vi "HFRR ADV v042.vi"() -> ()   [LabVIEW 2025] (continued)
        n1759 = Not Equal?(x=w2092, y=w2091) -> (x != y?=w2089:bool)
        n1760 = case shown="True" w2097 {
          frame False {
            w2103 = TRUE ("Visible")
            n1761 = property on="Port 1a" class="Bool (strict)"("Visible"=w2103) -> ()  [unwired: 2 in, 2 out]
            n1762 = property on="Port 3" class="Bool (strict)"("Visible"=w2103) -> ()  [unwired: 2 in, 2 out]
          }
          frame True {
            w2104 = TRUE ("Visible")
            n1763 = property on="Port 1a" class="Bool (strict)"("Visible"=w2104) -> ()  [unwired: 2 in, 2 out]
            n1764 = property on="Port 3" class="Bool (strict)"("Visible"=w2104) -> ()  [unwired: 2 in, 2 out]
          }
        }
        n1765 = Wait (ms)(milliseconds to wait=u32 40) -> ()  [unwired: 1 out]
        n1766 = case shown="True" w2089 {
          tunnel: [w2101 errorcluster {"status"=TRUE, "code"=0, "source"="Init"} ("error out")] -> w2090
          tunnel: w2093 -> [w2101 _]
          frame False {
          }
          frame True {
          }
        }
        n1767 = case shown="Error" w2090 {
          selector: w2090 -> [w2111 w2129]
          tunnel: [w2114 w2133] -> w2100
          tunnel: [w2113 w2127] -> w2099
          tunnel: w2091 -> [w2112 w2131]
          frame No Error {
            n1768 = property class="Instr"(reference=w2112, error in=w2111) -> (reference out=w2109:refnum<visa-resource-name>, error out=w2110:errorcluster, "Serial Settings:Number of Bytes at Serial Port"=w2106:u32)
            n1769 = Greater?(x=w2106, y=u32 5) -> (0:w2105:bool)
            n1770 = Not(x=w2105) -> (.not. x?=→"Port 1a":bool)
            n1771 = while {
              tunnel: [w2122] -> w2113
              tunnel: [w2121] -> w2114
              tunnel: w2110 -> [w2120]
              tunnel: w2109 -> [w2119]
              stop <- TRUE stop-if-true
              n1772 = property class="Instr" props=["Serial Settings:Number of Bytes at Serial Port"](reference=w2119, error in=w2120) -> (reference out=w2124:refnum<visa-resource-name>, error out=w2123:errorcluster)  [unwired: 1 out]
              n1773 = VISA Read(VISA resource name=w2124, byte count=u32 50, error in (no error)=w2123) -> (VISA resource name out=w2121:refnum<visa-resource-name>, read buffer=w2116:string, error out=w2122:errorcluster)  [unwired: 1 out]
              n1774 = Wait (ms)(milliseconds to wait=u32 5) -> ()  [unwired: 1 out]
            }
          }
          frame Error {
            w2139 = u16 0 items=["None", "XON/XOFF", "RTS/CTS", "XON/XOFF & RTS/CTS", "DTR/DSR", "XON/XOFF & DTR/DSR"] ("flow control (0:none)  2")
            w2137 = u16 10 items=["1.0"=10, "1.5"=15, "2.0"=20] ("stop bits 2")
            w2135 = u16 0 items=["None", "Odd", "Even", "Mark", "Space"] ("parity 2")
            w2136 = u32 10000  # timeout (10sec)
            n1775 = VISA Close(VISA resource name=w2131, error in (no error)=w2129) -> (error out=w2132:errorcluster)
            n1776 = local write "Port 1a"(FALSE ("Port 1a")) -> ()
            n1777 = local read "Com Port 1"() -> (w2126:refnum<visa-resource-name>)
            n1778 = call <vilib>:"Clear Errors.vi"("error in (no error)"=w2132) -> ("error out"=w2130:errorcluster)  [unwired: 5 in, 1 out]
            n1779 = call-poly "VISA Configure Serial Port"("VISA resource name"=w2126, "timeout (10sec)"=w2136, "baud rate (9600)"=u32 250000 ("baud rate  2"), "data bits (8)"=u16 8 ("data bits  2"), "parity (0:none)"=w2135, "error in (no error)"=w2130, "stop bits (10: 1 bit)"=w2137, "flow control (0:none)"=w2139) -> ("VISA resource name out"=w2140:refnum<visa-resource-name>, "error out"=w2141:errorcluster)  [unwired: 6 in]
            n1780 = flat-sequence {
              tunnel: w2140 -> [w2143]
              tunnel: w2141 -> [w2142]
              tunnel: [w2143] -> w2133
              tunnel: [w2142] -> w2127
              frame #0 {
                n1781 = Wait (ms)(milliseconds to wait=u32 50) -> ()  [unwired: 1 out]
              }
            }
            "Residual Uno" <- ""
          }
        }
        n1782 = local read "Quit"() -> (w2088:bool)
        "Error Uno" <- w2093
      }
      n1783 = VISA Close(VISA resource name=w2086, error in (no error)=w2085) -> (error out=w2083:errorcluster)
      n1784 = call <vilib>:"Clear Errors.vi"("error in (no error)"=w2083) -> ()  [unwired: 5 in, 2 out]
    }
    frame Enabled {
    }
  }
  n1785 = while {
    stop <- w2154 stop-if-true
    # "V0OLTAGE TO STROKE (peice vise calibration)"
    n1786 = local read "LVDT MIN"() -> (w2146:dbl)
    n1787 = local read "LVDT Peak"() -> (w2145:dbl)
    n1788 = Wait (ms)(milliseconds to wait=u32 10) -> ()  [unwired: 1 out]
    n1789 = formula code="// Dynamic Parameterized Linear Interpolation Node\n// Inputs: vpp_val, voltages (Array), distances (Array)\n// Outputs: stroke\n\nint i = 0;\nint segments = 11; // 12 points make 11 interpolation segments\n\n// 1. Lower Boundary Clamp\nif (vpp_val <= voltages[0]) {\n    stroke = distances[0];\n}\n// 2. Upper Boundary Clamp\nelse if (vpp_val >= voltages[segments]) {\n    stroke = distances[segments];\n}\n// 3. Dynamic Segment Search Loop\nelse {\n    stroke = distances[0]; // Fallback baseline\n    for (i = 0; i < segments; i++) {\n        if (vpp_val >= voltages[i] && vpp_val <= voltages[i+1]) {\n            // Standard linear interpolation formula using array lookups\n            stroke = distances[i] + (vpp_val - voltages[i]) * (distances[i+1] - distances[i]) / (voltages[i+1] - voltages[i]);\n            break; // Segment found, safely exit the loop\n        }\n    }\n}"("vpp_val"=w2145, "voltages"="calibration values", "distances"="STROKE") -> ("stroke"=→"LVDT STROKE":dbl)
    n1790 = local read "Calibration Tare Value"() -> (w2150:dbl)
    n1791 = local read "Calibration Tare"() -> (w2148:bool)
    n1792 = Subtract(x=w2146, y=w2150) -> (x-y=→"LVDT STROKE  Calibration":dbl)
    n1793 = case shown="True" w2148 {
      selector: w2148 -> [_ w2156]
      tunnel: w2146 -> [_ w2157]
      frame False {
      }
      frame True {
        n1794 = Not(x=w2156) -> (.not. x?=w2155:bool)
        n1795 = local write "Calibration Tare"(w2155) -> ()
        "Calibration Tare Value" <- w2157
      }
    }
    n1796 = local read "Quit"() -> (w2154:bool)
  }
  n1797 = while {
    stop <- w2180 stop-if-true
    n1798 = local read "Due read"() -> (w2178:string)
    n1799 = call <vilib>:"High Resolution Polling Wait.vi"("seconds to wait"=0.02) -> ()  [unwired: 10 in, 1 out]
    n1800 = local read "Frictioin Force Raw"() -> (w2160:dbl)
    n1801 = Spreadsheet String To Array(delimiter (Tab)=";", format string="", spreadsheet string=w2178, array type (2D Dbl)=string[] []) -> (array=w2175:string[])
    n1802 = Fract/Exp String To Number(string=w2175) -> (number=w2174:dbl[])  [unwired: 3 in, 1 out]
    n1803 = call <vilib>:"Median Filter PtByPt.vi"("rank"=2, "x"=w2160) -> ("Filtered x"=→"Friction":dbl)  [unwired: 2 in, 1 out]
    n1804 = Index Array(array=w2174) -> (element #1=→"Sample Temperature":dbl, element #2=→"Target Sample Temperature":dbl, element #3=→"Current Duty Cycle":dbl, element #4=→"Ambient Temperature":dbl, element #5=→"Dac Status":dbl, element #6=→"Vpp":dbl, element #7=→"Active Error Code":dbl, element #8=→"Kp":dbl, element #9=→"Ki":dbl, element #10=→"Kd":dbl, element #11=→"SampleRaw":dbl, element #12=→"AmbRaw":dbl)  [unwired: 12 in]
    n1805 = local read "Quit"() -> (w2180:bool)
  }
  n1806 = while {
    shift-right: [w2194] -> w43
    shift-left: _ -> [w2186]
    shift-right: [w2181] -> w42
    shift-left: errorcluster {"status"=FALSE, "code"=0, "source"="Init"} ("error out") -> [w2188]
    tunnel: [w2183] -> w46
    tunnel: [w2193] -> _
    i -> [w2193]
    stop <- w2183 stop-if-true
    n1807 = local read "Com Port 2"() -> (w2187:refnum<visa-resource-name>)
    n1808 = local read "Port 2a"() -> (w2189:bool)
    n1809 = Unbundle(w2188) -> ("status"=→"Port 4":bool)  [unwired: 2 out]
    n1810 = call <vilib>:"High Resolution Polling Wait.vi"("seconds to wait"=0.02) -> ()  [unwired: 10 in, 1 out]
    n1811 = local read "Port 4"() -> (w2190:bool)
    n1812 = Not Equal?(x=w2187, y=w2186) -> (x != y?=w2185:bool)
    n1813 = Or(x=w2190, y=w2189) -> (x .or. y?=w2192:bool)
    n1814 = case shown="False" w2192 {
      frame False {
        w2197 = TRUE ("Visible")
        n1815 = property on="Port 2a" class="Bool (strict)"("Visible"=w2197) -> ()  [unwired: 2 in, 2 out]
        n1816 = property on="Port 4" class="Bool (strict)"("Visible"=w2197) -> ()  [unwired: 2 in, 2 out]
      }
      frame True {
        w2198 = TRUE ("Visible")
        n1817 = property on="Port 2a" class="Bool (strict)"("Visible"=w2198) -> ()  [unwired: 2 in, 2 out]
        n1818 = property on="Port 4" class="Bool (strict)"("Visible"=w2198) -> ()  [unwired: 2 in, 2 out]
      }
    }
    n1819 = case shown="True" w2185 {
      tunnel: [w2195 errorcluster {"status"=TRUE, "code"=0, "source"="Init"} ("error out")] -> w2184
      tunnel: w2188 -> [w2195 _]
      frame False {
      }
      frame True {
      }
    }
    n1820 = case shown="No Error" w2184 {
      selector: w2184 -> [w2211 w2242]
      tunnel: [w2204 w2247] -> w2194
      tunnel: [w2212 w2240] -> w2181
      tunnel: w2186 -> [w2213 w2245]
      frame No Error {
        n1821 = property class="Instr" props=["Serial Settings:Number of Bytes at Serial Port"](reference=w2213, error in=w2211) -> (reference out=w2205:refnum<visa-resource-name>, error out=w2210:errorcluster)  [unwired: 1 out]
        n1822 = while {
          tunnel: [w2221] -> w2206
          tunnel: [w2220] -> w2207
          tunnel: w2210 -> [w2219]
          tunnel: w2205 -> [w2218]
          tunnel: [w2217] -> _
          i -> [w2217]
          stop <- TRUE stop-if-true
          n1823 = property class="Instr" props=["Serial Settings:Number of Bytes at Serial Port"](reference=w2218, error in=w2219) -> (reference out=w2223:refnum<visa-resource-name>, error out=w2222:errorcluster)  [unwired: 1 out]
          n1824 = VISA Read(VISA resource name=w2223, byte count=u32 1000, error in (no error)=w2222) -> (VISA resource name out=w2220:refnum<visa-resource-name>, read buffer=→"Due read":string, error out=w2221:errorcluster)  [unwired: 1 out]
        }
        n1825 = local read "Due Write"() -> (w2203:string)
        n1826 = call <vilib>:"Trim Whitespace.vi"("string"=w2203) -> ("trimmed string"=w2202:string)  [unwired: 1 in]
        n1827 = Not Equal?(x=w2202, y="") -> (x != y?=w2208:bool)
        n1828 = VISA Flush I/O Buffer(VISA resource name=w2207) -> (VISA resource name out=w2200:refnum<visa-resource-name>, error out=→"error out 10":errorcluster)  [unwired: 2 in]
        n1829 = case shown="True" w2208 {
          tunnel: w2200 -> [w2225 w2230]
          tunnel: [w2225 w2234] -> w2204
          tunnel: w2206 -> [w2224 w2229]
          tunnel: [w2224 w2232] -> w2212
          tunnel: w2202 -> [_ w2228]
          tunnel: [_ w2231] -> _
          frame False {
            # "DATA  WRITE LOOP"
          }
          frame True {
            n1830 = Concatenate Strings(w2228, "\r\n") -> (w2227:string)
            n1831 = VISA Write(VISA resource name=w2230, write buffer=w2227, error in (no error)=w2229) -> (VISA resource name out=w2234:refnum<visa-resource-name>, return count=w2231:u32, error out=w2233:errorcluster)
            n1832 = flat-sequence {
              tunnel: w2233 -> [w2236]
              tunnel: [w2236] -> w2232
              frame #0 {
                n1833 = local write "Due Write"("" ("Command")) -> ()
                n1834 = Wait (ms)(milliseconds to wait=u32 5) -> ()  [unwired: 1 out]
              }
            }
          }
        }
        "Port 2a" <- TRUE ("Port 2a")
      }
      frame Error {
        w2253 = u16 0 items=["None", "XON/XOFF", "RTS/CTS", "XON/XOFF & RTS/CTS", "DTR/DSR", "XON/XOFF & DTR/DSR"] ("flow control (0:none)  2")
        w2251 = u16 10 items=["1.0"=10, "1.5"=15, "2.0"=20] ("stop bits 2")
        w2249 = u16 0 items=["None", "Odd", "Even", "Mark", "Space"] ("parity 2")
        w2250 = u32 10000  # timeout (10sec)
        n1835 = VISA Clear(VISA resource name=w2245, error in (no error)=w2242) -> (VISA resource name out=w2244:refnum<visa-resource-name>, error out=w2243:errorcluster)
        n1836 = VISA Close(VISA resource name=w2244, error in (no error)=w2243) -> (error out=w2246:errorcluster)
        n1837 = call <vilib>:"Clear Errors.vi"("error in (no error)"=w2246) -> ()  [unwired: 5 in, 2 out]
        n1838 = local write "Port 2a"(FALSE ("Port 2a")) -> ()
        n1839 = local read "Com Port 2"() -> (w2239:refnum<visa-resource-name>)
        "visa due" <- w2239
        n1840 = call-poly "VISA Configure Serial Port"("VISA resource name"=w2239, "timeout (10sec)"=w2250, "baud rate (9600)"=u32 250000 ("baud rate  2"), "data bits (8)"=u16 8 ("data bits  2"), "parity (0:none)"=w2249, "stop bits (10: 1 bit)"=w2251, "flow control (0:none)"=w2253) -> ("VISA resource name out"=w2254:refnum<visa-resource-name>, "error out"=w2255:errorcluster)  [unwired: 7 in]
        n1841 = flat-sequence {
          tunnel: w2254 -> [w2257]
          tunnel: w2255 -> [w2256]
          tunnel: [w2257] -> w2247
          tunnel: [w2256] -> w2240
          frame #0 {
            n1842 = Wait (ms)(milliseconds to wait=u32 50) -> ()  [unwired: 1 out]
          }
        }
        "Residual Due" <- ""
      }
    }
    "error out 9" <- w2181
    n1843 = local read "Quit"() -> (w2183:bool)
    "Error Due" <- w2188
  }
  n1844 = local write "FRICVALZ"(0.0 ("FRICVALZ")) -> ()
  n1845 = property on="RUN" class="Bool (strict)"("Visible"=TRUE) -> ()  [unwired: 2 in, 2 out]
  n1846 = while {
    tunnel: [w2272] -> _
    tunnel: [w2259] -> w56
    i -> [w2272]
    stop <- w2259 stop-if-true
    n1847 = local read "conststatus"() -> (w2263:dbl)
    n1848 = local read "Main Tab"() -> (w2261:T2)
    n1849 = local read "EDIT"() -> (w2278:bool)
    n1850 = local read "Rate"() -> (w2277:dbl)
    n1851 = case shown="True" w2278 {
      tunnel: [FALSE TRUE] -> _
      frame False {
      }
      frame True {
      }
    }
    n1852 = Equal?(x=w2261, y=T28."About" ("Main Tab")) -> (x = y?=w2270:bool)
    n1853 = Equal?(x=w2263, y=0.0) -> (x = y?=w2264:bool)
    n1854 = Divide(x=1.0, y=w2277) -> (x/y=w2273:dbl)
    "Time 2" <- w2273
    n1855 = case shown="True" w2264 {
      frame False {
      }
      frame True {
        # "C:\\WinDucom\\calibrate WO 2391.dcf"
        n1856 = local write "Lan flag"(22) -> ()
        n1857 = local write "conststatus"(10.0 ("rpm value : 2")) -> ()
        n1858 = String To Path(string="C:\\LAB-IQ\\calibrate WO 2465.dcf") -> (path=w2284:path)
        n1859 = Open/Create/Replace File "Open File"(file path (use dialog)=w2284) -> (refnum out=w2282:refnum<file>)  [unwired: 5 in, 2 out]
        n1860 = for {
          N: 23 -> [_]
          tunnel: w2282 -> [w2293]
          i -> [w2287]
          (unwired) TRUE ("line mode (F)")
          n1861 = Read from Text File "Read File"(file (use dialog)=w2293) -> (text=w2292:string)  [unwired: 3 in, 3 out]
          n1862 = Match Pattern(string=w2292, regular expression="]") -> (after substring=w2290:string)  [unwired: 1 in, 3 out]
          n1863 = String Subset(string=w2292, offset (0)=5, length (rest)=10 ("length (rest)")) -> (substring=w2285:string)
          n1864 = Fract/Exp String To Number(string=w2285) -> (number=w2286:dbl)  [unwired: 3 in, 1 out]
          n1865 = Match Pattern(string=w2290, regular expression="-") -> (before substring=w2288:string)  [unwired: 1 in, 3 out]
          n1866 = case shown="10" w2287 {
            tunnel: w2286 -> [_ _ _ _ _ _ _ _ _ _ w2300 _ _ _ _ _ _ _ _ _ _ _ _ _]
            tunnel: w2288 -> [_ _ _ _ w2296 w2297 w2298 _ _ _ _ _ _ _ _ _ _ _ _ _ w2301 w2302 w2303 _]
            frame 0 {
            }
            frame 1 {
            }
            frame 2 {
            }
            frame 3 {
            }
            frame 4 {
              n1867 = local write "Com Port 1"(w2296) -> ()
            }
            frame 5 {
              n1868 = local write "Com Port 2"(w2297) -> ()
              n1869 = local write "visa due"(w2297) -> ()
            }
            frame 6 {
              n1870 = String To Path(string=w2298) -> (path=w2299:path)
              n1871 = local write "File Path"(w2299) -> ()
              "String" <- w2298
            }
            frame 7 {
            }
            frame 8 {
            }
            frame 9 {
            }
            frame 10 {
              n1872 = local write "Language Selection"(w2300) -> ()
            }
            frame 11 {
            }
            frame 12 {
            }
            frame 13 {
            }
            frame 14 {
            }
            frame 15 {
            }
            frame 16 {
            }
            frame 17 {
            }
            frame 18 {
            }
            frame 21 {
            }
            frame 22 {
              n1873 = local write "Com Port 3"(w2301) -> ()
            }
            frame 20 {
              n1874 = local write "Camera Port :"(w2302) -> ()
            }
            frame 19 {
              n1875 = local write "C3 :"(w2303) -> ()
            }
            frame 23, Default {
            }
          }
        }
      }
    }
    n1876 = Select(t=u32 2500 ("milliseconds to wait"), s=w2270, f=u32 500 ("milliseconds to wait")) -> (s? t:f=w2268:u32)
    n1877 = Multiply(x=w2273, y=w2268) -> (x*y=w2275:dbl)
    n1878 = call "Elapsed Time2"("Time Target (s)"=w2275, "Auto Reset"=TRUE) -> ("Time has Elapsed"=w2265:bool)  [unwired: 10 in, 7 out]
    n1879 = case shown="True" w2265 {
      frame False {
      }
      frame True {
        n1880 = stacked-sequence {
          frame #0 {
            # "DATA PROCESSING"
            # "115 mV/N"
            n1881 = local read "Sample Temperature"() -> (w2306:dbl)
            n1882 = local read "RH Numeric:"() -> (→"Humidity ( %RH )":dbl)
            n1883 = local read "FRICVALZ"() -> (w2323:dbl)
            n1884 = local read "Friction"() -> (w2309:dbl)
            n1885 = call <vilib>:"Mean PtByPt.vi"("x"=w2306, "sample length"=100) -> ("mean"=w2305:dbl)  [unwired: 2 in, 1 out]
            "TEMP 2" <- w2305
            "TEMP 3" <- w2305
            n1886 = Subtract(x=w2309, y=w2323) -> (x-y=w2318:dbl)
            "FF 2" <- w2318
            "FF 4" <- w2318
            n1887 = local read "Ambient Temperature"() -> (→"AIR TEMP":dbl)
            n1888 = local read "TEMP"() -> (w2322:dbl)
            n1889 = local write "FF 3"(w2318) -> ()
            n1890 = Compound Arithmetic op=OR("FRICVALZ 4", "FRICVALZ 3", "FRICVALZ 2") -> (w2314:bool)
            n1891 = case shown="True" w2314 {
              tunnel: w2309 -> [_ w2329]
              frame False {
              }
              frame True {
                w2328 = FALSE ("FRICVALZ")
                n1892 = local write "FRICVALZ 3"(w2328) -> ()
                n1893 = local write "FRICVALZ 2"(w2328) -> ()
                n1894 = local write "FRICVALZ 4"(w2328) -> ()
                "FRICVALZ" <- w2329
              }
            }
            n1895 = Not A Number/Path/Refnum?(number/path/refnum=w2322) -> (NaN/Path/Refnum?=w2321:bool)
            n1896 = Not A Number/Path/Refnum?(number/path/refnum=w2318) -> (NaN/Path/Refnum?=w2320:bool)
            n1897 = Divide(x=w2318, y=1.96) -> (x/y=w2315:dbl)
            n1898 = Compound Arithmetic op=OR(w2321, w2320) -> (w2319:bool)
            n1899 = Not A Number/Path/Refnum?(number/path/refnum=w2315) -> (NaN/Path/Refnum?=w2316:bool)
            n1900 = case shown="True" w2319 {
              frame False {
              }
              frame True {
                n1901 = local write "TEMP"(0.0 ("TEMP")) -> ()
                n1902 = local write "FF 2"(0.0 ("FF 2")) -> ()
                n1903 = local write "reinit"(TRUE ("reinit")) -> ()
              }
            }
            n1904 = local write "TEMP"(w2305) -> ()
            n1905 = Select(t=0.0, s=w2316, f=w2315) -> (s? t:f=w2308:dbl)
            "COF 2" <- w2308
            n1906 = local write "COF 3"(w2308) -> ()
          }
        }
      }
    }
    n1907 = Wait (ms)(milliseconds to wait=u32 50) -> ()  [unwired: 1 out]
    n1908 = local read "Quit"() -> (w2259:bool)
    "Rate" <- 2500.0 ("No of Samples")
  }
  n1909 = while {
    tunnel: [w2349] -> _
    tunnel: [w2332] -> w58
    tunnel: w3 -> [_]
    i -> [w2349]
    stop <- w2332 stop-if-true
    # "C:\\LAB-IQ-NXT\\Scar View.exe"
    n1910 = local read "OK Button 16"() -> (w2339:bool)
    n1911 = local read "Main Tab"() -> (w2333:T2)
    n1912 = local read "service 3"() -> (w2334:bool)
    n1913 = local read "OPEN 6"() -> (w2336:bool)
    n1914 = local read "EDIT 2"() -> (w2338:bool)
    n1915 = flat-sequence {
      frame #0 {
        n1916 = stacked-sequence {
          frame #0 {
            n1917 = local read "EDIT"() -> (w2827:bool)
            n1918 = case shown="False" w2827 {
              tunnel: [u8 2 ("Disabled") u8 0 ("Disabled")] -> _
              frame False {
                w2829 = FALSE
                n1919 = local write "Password"("") -> ()
                n1920 = local write "x = y?"(w2829) -> ()
                n1921 = property on="Password" class="Str"("Visible"=w2829) -> ()  [unwired: 2 in, 2 out]
              }
              frame True {
                n1922 = property on="Password" class="Str"("Visible"=TRUE) -> ()  [unwired: 2 in, 2 out]
              }
            }
            "dipl pwd" <- "@143$\n" ("dipl pwd")
          }
          frame #1 {
          }
          frame #2 {
          }
          frame #3 {
          }
          frame #4 {
            n1923 = String To Byte Array(string="Password") -> (unsigned byte array=w2840:u8[])
            n1924 = Search 1D Array(1D array=w2840, element=u8 10) -> (index of element=w2838:i32)  [unwired: 1 in]
            n1925 = Index Array(array=w2840, index=w2838) -> (element=w2839:u8)
            n1926 = Equal?(x=w2839, y=10) -> (x = y?=w2835:bool)
            n1927 = case shown="True" w2835 {
              frame False {
              }
              frame True {
                # "password"
                # "password"
                n1928 = local read "Password"() -> (w2852:string)
                n1929 = String To Byte Array(string=w2852) -> (unsigned byte array=w2855:u8[])
                n1930 = String To Byte Array(string="@143$\n") -> (unsigned byte array=w2842:u8[])
                n1931 = Array Size(array=w2855) -> (size(s)=w2851:i32)
                n1932 = Array Size(array=w2842) -> (size(s)=w2847:i32)
                n1933 = for {
                  N: w2851 -> [_]
                  tunnel: w2855 -> [w2868]
                  tunnel: [w2866] -> w2856 mode=indexing
                  tunnel: w2851 -> [w2863]
                  i -> [w2864]
                  n1934 = Decrement(x=w2863) -> (x-1=w2862:i32)
                  n1935 = Index Array(array=w2868, index=w2864) -> (element=w2867:u8)
                  n1936 = Equal?(x=w2864, y=w2862) -> (x = y?=w2861:bool)
                  n1937 = Number To Decimal String(number=w2867) -> (decimal integer string=w2865:string)  [unwired: 1 in]
                  n1938 = Select(t="", s=w2861, f="\r") -> (s? t:f=w2858:string)
                  n1939 = Concatenate Strings(w2865, w2858) -> (w2866:string)
                }
                n1940 = for {
                  N: w2847 -> [_]
                  tunnel: w2842 -> [w2879]
                  tunnel: [w2877] -> w2845 mode=indexing
                  tunnel: w2847 -> [w2874]
                  i -> [w2875]
                  n1941 = Decrement(x=w2874) -> (x-1=w2873:i32)
                  n1942 = Index Array(array=w2879, index=w2875) -> (element=w2878:u8)
                  n1943 = Equal?(x=w2875, y=w2873) -> (x = y?=w2872:bool)
                  n1944 = Number To Decimal String(number=w2878) -> (decimal integer string=w2876:string)  [unwired: 1 in]
                  n1945 = Select(t="", s=w2872, f="\r") -> (s? t:f=w2869:string)
                  n1946 = Concatenate Strings(w2876, w2869) -> (w2877:string)
                }
                n1947 = local read "file path"() -> (w2841:path)
                n1948 = call <vilib>:"Read Characters From File.vi"("file path (dialog if empty)"=w2841) -> ("character string"=w2854:string)  [unwired: 5 in, 3 out]
                "string" <- w2854
                n1949 = flat-sequence {
                  tunnel: [w2857] -> _
                  frame #0 {
                    w2857 = ""
                    n1950 = local write "Password"(w2857) -> ()
                  }
                }
                n1951 = Concatenate Strings(w2845) -> (w2846:string)
                n1952 = Concatenate Strings(w2854) -> (w2853:string)
                n1953 = Concatenate Strings(w2856) -> (w2849:string)
                n1954 = Equal?(x=w2849, y=w2853) -> (x = y?=w2844:bool)
                n1955 = Equal?(x=w2849, y=w2846) -> (x = y?=w2850:bool)
                n1956 = Or(x=w2844, y=w2850) -> (x .or. y?=→"x = y?":bool)
              }
            }
          }
        }
        n1957 = local read "x = y?"() -> (w2825:bool)
        n1958 = And(x="EDIT", y=w2825) -> (x .and. y?=w2823:bool)
        n1959 = case shown="True" w2823 {
          tunnel: [u8 2 ("Disabled") u8 0 ("Disabled")] -> w2822
          tunnel: [w3029 TRUE ("Visible")] -> w2821
          frame False {
            w3029 = FALSE ("Visible")
            n1960 = local write "EDIT 2"(w3029) -> ()
          }
          frame True {
          }
        }
        n1961 = case shown="True" "SAVE" {
          frame False {
          }
          frame True {
            n1962 = stacked-sequence {
              seq-local: [w2884 _ _] -> [_ w3025 _]
              frame #0 {
                w2880 = 0.0 ("number")
                w2881 = 0.0 ("number")
                (unwired) i16 5 ("precision (6)")
                # "[CH1]    - FF\n[CH2]   - TEMPERATURE\n[CH3]    - Humidity\n[CH4]    - AIR TEMP\n[CH5]\\- Visa Uno\n[CH6] \\- Visa Due\n[CH7]  \\- file path\n[CH8]   - Displacement Gain\n[CHA]   - Stroke Gain\n[CHB]   - Stroke PID Gain\n[CHC]   -Language Selection\n[CHD]   -Power +\n[CHE]   -Power_\n[CHF]   -Heater\n[CHG]   -Humidity Wet\n[CHH]   -Humidity Dry\n[CHI]   -Integral Time"
                n1963 = local read "Language Selection"() -> (w2927:enum16{"English", "Russian"})
                n1964 = Path To String(path="File Path") -> (string=w2943:string)
                n1965 = Number To Fractional String(number=w2880, width (-)=i16 10 ("precision (6)"), precision (6)=i16 5) -> (F-format string=w2934:string)  [unwired: 1 in]
                n1966 = Number To Fractional String(number=w2927, width (-)=i16 10 ("precision (6)"), precision (6)=i16 5) -> (F-format string=w2923:string)  [unwired: 1 in]
                n1967 = Number To Fractional String(number=w2881, width (-)=i16 10 ("precision (6)"), precision (6)=i16 5) -> (F-format string=w2917:string)  [unwired: 1 in]
                n1968 = Number To Fractional String(number=w2881, width (-)=i16 10 ("precision (6)"), precision (6)=i16 5) -> (F-format string=w2914:string)  [unwired: 1 in]
                n1969 = Number To Fractional String(number=w2881, width (-)=i16 10 ("precision (6)"), precision (6)=i16 5) -> (F-format string=w2909:string)  [unwired: 1 in]
                n1970 = Number To Fractional String(number=w2881, width (-)=i16 10 ("precision (6)"), precision (6)=i16 5) -> (F-format string=w2906:string)  [unwired: 1 in]
                n1971 = Number To Fractional String(number=w2881, width (-)=i16 10 ("precision (6)"), precision (6)=i16 5) -> (F-format string=w2901:string)  [unwired: 1 in]
                n1972 = local read "Com Port 1"() -> (w2883:refnum<visa-resource-name>)
                n1973 = local read "Com Port 2"() -> (w2882:refnum<visa-resource-name>)
                n1974 = Concatenate Strings(w2943, "\\" ("string")) -> (w2942:string)
                n1975 = Number To Fractional String(number=w2880, width (-)=i16 10 ("precision (6)"), precision (6)=i16 5) -> (F-format string=w2975:string)  [unwired: 1 in]
                n1976 = Number To Fractional String(number=w2880, width (-)=i16 10 ("precision (6)"), precision (6)=i16 5) -> (F-format string=w2974:string)  [unwired: 1 in]
                n1977 = Number To Fractional String(number=w2880, width (-)=i16 10 ("precision (6)"), precision (6)=i16 5) -> (F-format string=w2968:string)  [unwired: 1 in]
                n1978 = Number To Fractional String(number=w2880, width (-)=i16 10 ("precision (6)"), precision (6)=i16 5) -> (F-format string=w2962:string)  [unwired: 1 in]
                n1979 = Number To Fractional String(number=w2880, width (-)=i16 10 ("precision (6)"), precision (6)=i16 5) -> (F-format string=w2935:string)  [unwired: 1 in]
                n1980 = Concatenate Strings("[CHA]" ("string"), w2934, "- Stroke Gain" ("string"), "\r") -> (w2928:string)
                n1981 = Concatenate Strings("[CHC]" ("string"), w2923, "-Language Selection" ("string"), "\r") -> (w2920:string)
                n1982 = Concatenate Strings("[CHD]" ("string"), w2917, "-Power +" ("string"), "\r") -> (w2899:string)
                n1983 = Concatenate Strings("[CHG]" ("string"), w2906, "-Humidity Wet" ("string"), "\r") -> (w2896:string)
                n1984 = Concatenate Strings("[CHH]" ("string"), w2901, "-Humidity Dry" ("string"), "\r") -> (w2895:string)
                n1985 = Concatenate Strings("[CH1]" ("string"), w2975, " - FF" ("string"), "\r") -> (w2973:string)
                n1986 = Concatenate Strings("[CH2]" ("string"), w2974, " - TEMPERATURE" ("string"), "\r") -> (w2972:string)
                n1987 = Concatenate Strings("[CH3]" ("string"), w2968, " - Humidity" ("string"), "\r") -> (w2965:string)
                n1988 = Concatenate Strings("[CH4]" ("string"), w2962, " - AIR TEMP" ("string"), "\r") -> (w2958:string)
                n1989 = Concatenate Strings("[CH5]" ("string"), w2883, "- Visa Uno" ("string"), "\r") -> (w2951:string)
                n1990 = Concatenate Strings("[CH6]" ("string"), w2882, "- Visa Due" ("string"), "\r") -> (w2946:string)
                n1991 = Concatenate Strings("[CH7]" ("string"), w2942, "- file path" ("string"), "\r") -> (w2945:string)
                n1992 = Concatenate Strings("[CH8]" ("string"), w2935, "- Displacement Gain" ("string"), "\r") -> (w2938:string)
                n1993 = Concatenate Strings("[CHE]" ("string"), w2914, "-Power_" ("string"), "\r") -> (w2898:string)
                n1994 = Concatenate Strings("[CHF]" ("string"), w2909, "-Heater" ("string"), "\r") -> (w2897:string)
                n1995 = Concatenate Strings(w2973, w2972, w2965, w2958, w2951, w2946, w2945, w2938, w2928, w2920, w2899, w2898, w2897, w2896, w2895) -> (w2884:string)
                "gain" <- w2884
              }
              frame #1 {
                w2986 = 0.0 ("number")
                n1996 = local read "Camera Port :"() -> (w2989:string)
                n1997 = local read "C3 :"() -> (w2997:refnum<visa-resource-name>)
                n1998 = local read "Com Port 3"() -> (w2998:refnum<visa-resource-name>)
                n1999 = Concatenate Strings("[CH8]" ("string"), w2989, "- Visa Camera" ("string"), "\r") -> (w2988:string)
                n2000 = Concatenate Strings("[CH7]" ("string"), w2997, "- Visa Humidity" ("string"), "\r") -> (w2993:string)
                n2001 = Number To Fractional String(number=w2986, width (-)=i16 10 ("precision (6)"), precision (6)=i16 5) -> (F-format string=w3013:string)  [unwired: 1 in]
                n2002 = Concatenate Strings("[CHL]" ("string"), w2998, "- Visa humid" ("string"), "\r") -> (w3001:string)
                n2003 = Number To Fractional String(number=w2986, width (-)=i16 10 ("precision (6)"), precision (6)=i16 5) -> (F-format string=w3020:string)  [unwired: 1 in]
                n2004 = Concatenate Strings("[CHK]" ("string"), w3013, "-TEMP INTERCEPT" ("string"), "\r") -> (w3009:string)
                n2005 = Concatenate Strings("[SNO]" ("string"), "" ("string"), "-" ("string"), "\r") -> (w3006:string)
                n2006 = Concatenate Strings("[CHJ]" ("string"), w3020, "-AIR TEMP INTERCEPT" ("string"), "\r") -> (w3010:string)
                n2007 = String To Path(string="C:\\LAB-IQ\\calibrate WO 2465.dcf") -> (path=w2999:path)
                n2008 = Concatenate Strings(w3025, w3010, w3009, w3006, w3001, w2993, w2988) -> (w3024:string)
                n2009 = call <vilib>:"Write Characters To File.vi"("append to file? (new file:F)"=FALSE, "character string"=w3024, "file path (dialog if empty)"=w2999) -> ()  [unwired: 2 in, 1 out]
              }
              frame #2 {
                n2010 = local write "Lan flag"(0.0 ("Lan flag")) -> ()
                n2011 = local write "conststatus"(0.0 ("rpm value : 2")) -> ()
                n2012 = local write "SAVE"(FALSE ("OK Button 14")) -> ()
              }
            }
          }
        }
        n2013 = property on="EDIT 2" class="Bool (strict)"("Visible"=w2821) -> ()  [unwired: 2 in, 2 out]
        n2014 = property on="SAVE" class="Bool (strict)"("Visible"=w2821) -> ()  [unwired: 2 in, 2 out]
        n2015 = property on="visa due" class="CmbBox"("Disabled"=w2822) -> ()  [unwired: 2 in, 2 out]
        n2016 = property on="File Path" class="Path"("Disabled"=w2822) -> ()  [unwired: 2 in, 2 out]
        n2017 = property on="Language Selection" class="Enum (strict)"("Visible"=w2821) -> ()  [unwired: 2 in, 2 out]
        n2018 = property on="SPEED OUT:" class="DigNum (strict)"("Disabled"=w2822) -> ()  [unwired: 2 in, 2 out]
      }
    }
    n2019 = local read "RUN"() -> (w2348:bool)
    n2020 = local read "RUN"() -> (w2346:bool)
    n2021 = case shown="True" "EDIT 3" {
      frame False {
      }
      frame True {
        n2022 = local write "EDIT 3"(FALSE ("EDIT 3")) -> ()
        n2023 = local write "Main Tab"(T2."About" ("Main Tab")) -> ()
      }
    }
    n2024 = case shown="False" w2348 {
      frame False {
        n2025 = local read "stopT"() -> (w3036:bool)
        n2026 = case shown="True" w3036 {
          frame False {
          }
          frame True {
            n2027 = local write "stopT"(FALSE) -> ()
          }
        }
      }
      frame True {
        "stopT" <- TRUE
      }
    }
    n2028 = case shown="False" w2346 {
      frame False {
      }
      frame True {
      }
    }
    n2029 = case shown="True" w2338 {
      frame False {
        n2030 = property on="Password 2" class="Str"("Visible"=FALSE) -> ()  [unwired: 2 in, 2 out]
        n2031 = local write "Password 2"("" ("Password")) -> ()
      }
      frame True {
        n2032 = property on="Password 2" class="Str"("Visible"=TRUE) -> ()  [unwired: 2 in, 2 out]
        n2033 = Equal?(x="Password 2", y="HFRR1234") -> (x = y?=w2361:bool)
        n2034 = case shown="True" w2361 {
          tunnel: "Password 2" -> [w2364 _]
          frame False {
            n2035 = String Length(string=w2364) -> (length=w2365:i32)
            n2036 = Greater Than 0?(x=w2365) -> (x > 0?=w2363:bool)
            n2037 = case shown="False" w2363 {
              frame False {
                n2038 = property on="Password 2" class="Str"("Caption.Text"="Password (Advance Setting)") -> ()  [unwired: 2 in, 2 out]
              }
              frame True {
                n2039 = property on="Password 2" class="Str"("Caption.Text"="Incorrect Password!") -> ()  [unwired: 2 in, 2 out]
              }
            }
          }
          frame True {
            n2040 = local write "EDIT 2"(FALSE ("EDIT 2")) -> ()
            n2041 = local write "Password 2"("" ("Password")) -> ()
            n2042 = local write "Main Tab"(T2."Advance" ("Main Tab")) -> ()
            n2043 = local write "Main Dashboard Buttons"(T1."Advance" ("Main Dashboard Buttons")) -> ()
          }
        }
      }
    }
    n2044 = case shown="True" "Prog Uno" {
      frame False {
      }
      frame True {
        n2045 = stacked-sequence {
          frame #0 {
            n2046 = Delete(path (use dialog)=path "C:/LAB-IQ-NXT/UNOCOMPILE.bat" ("working directory")) -> ()  [unwired: 4 in, 3 out]
          }
          frame #1 {
            n2047 = local read "Com Port 1"() -> (w2803:refnum<visa-resource-name>)
            n2048 = Concatenate Strings("cmd.exe /c \"mode " ("command line"), w2803, ":1200,n,8,1\"\n" ("command line")) -> (w2808:string)
            n2049 = Concatenate Strings(w2808, "CD\\\nCD WinDucom\navrdude -C avrdude.conf -v -patmega328p -carduino -P" ("command line"), w2803, " -b115200 -D -Uflash:w:UNO_V20.hex:i\n" ("command line"), "\r") -> (w2810:string)
            "STR" <- w2810
            n2050 = call <vilib>:"Write Characters To File.vi"("append to file? (new file:F)"=FALSE, "character string"=w2810, "file path (dialog if empty)"=path "C:/LAB-IQ/UNOCOMPILE.bat" ("working directory")) -> ()  [unwired: 2 in, 1 out]
          }
          frame #2 {
            n2051 = disable-structure shown="Disabled" {
              frame Disabled {
                w2814 = "cmd.exe  /c \"C:\\LAB-IQ-NXT\\UNOCOMPILE.bat\"" ("string")
                n2052 = local write "Prog Uno"(FALSE ("run minimized? (F)")) -> ()
                n2053 = call <vilib>:"System Exec.vi"("expected output size  (4096)"=u32 65535, "run minimized? (F)"=FALSE, "wait until completion? (T)"=TRUE ("run minimized? (F)"), "working directory"=path "C:/LAB-IQ-NXT", "standard input"=w2814, "command line"=w2814) -> ("error out"=w2813:errorcluster, "standard output"=→"String 42":string)  [unwired: 2 in, 2 out]
                "error out 3" <- w2813
                n2054 = flat-sequence {
                  tunnel: w2813 -> [_]
                  frame #0 {
                  }
                }
              }
              frame Enabled {
              }
            }
          }
        }
      }
    }
    n2055 = case shown="\"ISO 12156\"" "TEST STANDARD" {
      frame "ASTM D6079", Default {
        w2783 = 50.0 ("Hz")
        w2784 = 53.0 ("Set Rh")
        w2786 = 1.0 ("Set Strk")
        w2785 = 60.0 ("Set Temp")
        # "astm hide"
        n2056 = local write "NORMAL LOAD"(200.0 ("NORMAL LOAD")) -> ()
        n2057 = local write "Set Strk"(w2786) -> ()
        n2058 = local write "Set Hz"(w2783) -> ()
        n2059 = local write "Set Temp"(w2785) -> ()
        n2060 = local write "Set Rh"(w2784) -> ()
        n2061 = local write "test time"(75.0 ("test time")) -> ()
        n2062 = local write "Set Stroke:"(w2786) -> ()
        n2063 = local write "Set Humidity:"(w2784) -> ()
        n2064 = local write "Set Frequency:"(w2783) -> ()
        n2065 = local write "Set Temperature:"(w2785) -> ()
        "Test Standard" <- "ASTM D6079" ("Test Standard 2")
      }
      frame "ISO 12156" {
        n2066 = local write "Set Strk"(1.0 ("Set Strk")) -> ()
        n2067 = local write "NORMAL LOAD"(200.0 ("NORMAL LOAD")) -> ()
        n2068 = local write "Set Temp"(60.0 ("Set Temp")) -> ()
        n2069 = local write "test time"(75.0 ("test time")) -> ()
        n2070 = local write "Set Hz"(50.0 ("Hz")) -> ()
        n2071 = local write "Set Rh"(53.0 ("Set Rh")) -> ()
      }
      frame "CEC F-096-A-06" {
        n2072 = local write "Set Strk"(1.0 ("Set Strk")) -> ()
        n2073 = local write "NORMAL LOAD"(200.0 ("NORMAL LOAD")) -> ()
        n2074 = local write "Set Temp"(60.0 ("Set Temp")) -> ()
        n2075 = local write "test time"(75.0 ("test time")) -> ()
        n2076 = local write "Set Hz"(50.0 ("Hz")) -> ()
        n2077 = local write "Set Rh"(53.0 ("Set Rh")) -> ()
      }
      frame "Custom" {
      }
    }
    n2078 = Or(x=w2336, y=w2334) -> (x .or. y?=w2335:bool)
    n2079 = case shown="\"About\"" w2333 {
      tunnel: [T28."Acquire" ("Main Tab") T28."Compare Files" ("Main Tab") T28."About" ("Main Tab")] -> w2344
      frame "Acquire", Default {
      }
      frame "Compare Files" {
      }
      frame "About" {
      }
    }
    n2080 = Or(x=w2339, y="OPEN") -> (x .or. y?=w2340:bool)
    n2081 = case shown="True" w2340 {
      tunnel: w2339 -> [_ w2372]
      frame False {
      }
      frame True {
        n2082 = stacked-sequence {
          tunnel: w2372 -> [_ w2439 _ _]
          frame #0 {
            w2388 = "  " ("String 6")
            n2083 = local write "OPEN"(FALSE ("open")) -> ()
            n2084 = local read "string1 2"() -> (w2376:string)
            n2085 = local read "string1 3"() -> (w2375:string)
            n2086 = local read "string1 4"() -> (w2374:string)
            n2087 = property on="OPEN" class="Bool (strict)"("Visible"=FALSE) -> ()  [unwired: 2 in, 2 out]
            n2088 = local write "String 6"(w2388) -> ()
            n2089 = local write "String 7"(w2388) -> ()
            n2090 = local write "String 8"(w2388) -> ()
            n2091 = local write "String 12"(w2388) -> ()
            n2092 = local read "OK Button 16"() -> (w2373:bool)
            n2093 = String To Path(string=w2376) -> (path=w2384:path)
            n2094 = String To Path(string=w2375) -> (path=w2383:path)
            n2095 = String To Path(string=w2374) -> (path=w2382:path)
            n2096 = case shown="True" w2373 {
              tunnel: [w2389 w2390] -> w2377
              frame False {
                n2097 = local read "string1"() -> (w2389:string)
              }
              frame True {
                n2098 = local read "String Indicator 4"() -> (w2390:string)
              }
            }
            n2099 = Open/Create/Replace File "Open File"(file path (use dialog)=w2384) -> (refnum out=w2380:refnum<file>)  [unwired: 5 in, 2 out]
            n2100 = Open/Create/Replace File "Open File"(file path (use dialog)=w2383) -> (refnum out=w2379:refnum<file>)  [unwired: 5 in, 2 out]
            n2101 = Open/Create/Replace File "Open File"(file path (use dialog)=w2382) -> (refnum out=w2378:refnum<file>)  [unwired: 5 in, 2 out]
            n2102 = while {
              tunnel: w2380 -> [w2402]
              i -> [w2398]
              stop <- w2397 continue-if-true
              (unwired) TRUE ("line mode (F)")
              n2103 = Read from Text File "Read File"(file (use dialog)=w2402) -> (text=w2399:string)  [unwired: 3 in, 3 out]
              n2104 = local write "Numeric 11"(w2398) -> ()
              n2105 = String Length(string=w2399) -> (length=w2401:i32)
              n2106 = Greater?(x=w2401, y=1) -> (0:w2397:bool)
            }
            n2107 = while {
              tunnel: w2379 -> [w2408]
              i -> [w2404]
              stop <- w2403 continue-if-true
              (unwired) TRUE ("line mode (F)")
              n2108 = Read from Text File "Read File"(file (use dialog)=w2408) -> (text=w2405:string)  [unwired: 3 in, 3 out]
              n2109 = local write "Numeric 12"(w2404) -> ()
              n2110 = String Length(string=w2405) -> (length=w2407:i32)
              n2111 = Greater?(x=w2407, y=1) -> (0:w2403:bool)
            }
            n2112 = while {
              tunnel: w2378 -> [w2414]
              i -> [w2410]
              stop <- w2409 continue-if-true
              (unwired) TRUE ("line mode (F)")
              n2113 = Read from Text File "Read File"(file (use dialog)=w2414) -> (text=w2411:string)  [unwired: 3 in, 3 out]
              n2114 = local write "Numeric 13"(w2410) -> ()
              n2115 = String Length(string=w2411) -> (length=w2413:i32)
              n2116 = Greater?(x=w2413, y=1) -> (0:w2409:bool)
            }
            n2117 = String To Path(string=w2377) -> (path=w2385:path)
            n2118 = Open/Create/Replace File "Open File"(file path (use dialog)=w2385) -> (refnum out=w2381:refnum<file>)  [unwired: 5 in, 2 out]
            n2119 = while {
              tunnel: w2381 -> [w2396]
              i -> [w2392]
              stop <- w2391 continue-if-true
              (unwired) TRUE ("line mode (F)")
              n2120 = Read from Text File "Read File"(file (use dialog)=w2396) -> (text=w2393:string)  [unwired: 3 in, 3 out]
              n2121 = local write "Numeric 8"(w2392) -> ()
              n2122 = String Length(string=w2393) -> (length=w2395:i32)
              n2123 = Greater?(x=w2395, y=1) -> (0:w2391:bool)
            }
          }
          frame #1 {
            w2566 = FALSE ("ACTUAL   MERGE")
            # "Sample Temp"
            # "ECR"
            # "COF"
            # "Time\nCOF\nFF\nTemp"
            n2124 = case shown="True" w2439 {
              tunnel: [w2586 w2587] -> w2440
              frame False {
                n2125 = local read "string1"() -> (w2586:string)
              }
              frame True {
                n2126 = local read "String Indicator 4"() -> (w2587:string)
              }
            }
            n2127 = local read "string1 3"() -> (w2484:string)
            n2128 = String To Path(string=w2440) -> (path=w2571:path)
            n2129 = String To Path(string=w2484) -> (path=w2582:path)
            n2130 = local read "Numeric 12"() -> (w2568:i32)
            n2131 = local read "Numeric 8"() -> (w2570:i32)
            n2132 = local read "string1 2"() -> (w2485:string)
            n2133 = local read "string1 4"() -> (w2483:string)
            n2134 = Open/Create/Replace File "Open File"(file path (use dialog)=w2571) -> (refnum out=w2585:refnum<file>, error out=w2584:errorcluster)  [unwired: 5 in, 1 out]
            n2135 = Open/Create/Replace File "Open File"(file path (use dialog)=w2582) -> (refnum out=w2578:refnum<file>, error out=w2579:errorcluster)  [unwired: 5 in, 1 out]
            n2136 = for {
              N: w2570 -> [_]
              tunnel: w2585 -> [w2733]
              tunnel: w2584 -> [w2732]
              tunnel: [w2722] -> w2497 mode=indexing
              tunnel: [w2720] -> w2554 mode=indexing
              tunnel: [w2721] -> w2549 mode=indexing
              tunnel: w2566 -> [_]
              tunnel: [w2714] -> w2551 mode=indexing
              tunnel: [w2710] -> w2520 mode=indexing
              tunnel: [w2706] -> w2495 mode=indexing
              tunnel: [w2702] -> w2476 mode=indexing
              tunnel: [w2697] -> w2436 mode=indexing
              (unwired) TRUE ("line mode (F)")
              # "freq"
              # "Stroke"
              # "Time"
              # "CoF"
              # "Humidity"
              # "Temp"
              # "Air Temp"
              # "ECR"
              n2137 = Read from Text File "Read File"(file (use dialog)=w2733, error in=w2732) -> (text=w2698:string)  [unwired: 2 in, 3 out]
              n2138 = local write "String 6"(w2698) -> ()
              n2139 = String Subset(string=w2698, offset (0)=0, length (rest)=14 ("length (rest)")) -> (substring=w2726:string)
              n2140 = String Subset(string=w2698, offset (0)=35, length (rest)=9 ("length (rest)")) -> (substring=w2723:string)
              n2141 = String Subset(string=w2698, offset (0)=15, length (rest)=9 ("length (rest)")) -> (substring=w2729:string)
              n2142 = Fract/Exp String To Number(string=w2726) -> (number=w2722:dbl)  [unwired: 3 in, 1 out]
              n2143 = Fract/Exp String To Number(string=w2723) -> (number=w2721:dbl)  [unwired: 3 in, 1 out]
              n2144 = Fract/Exp String To Number(string=w2729) -> (number=w2720:dbl)  [unwired: 3 in, 1 out]
              n2145 = String Subset(string=w2698, offset (0)=85, length (rest)=9 ("length (rest)")) -> (substring=w2699:string)
              n2146 = String Subset(string=w2698, offset (0)=25, length (rest)=9 ("length (rest)")) -> (substring=w2705:string)
              n2147 = String Subset(string=w2698, offset (0)=55, length (rest)=9 ("length (rest)")) -> (substring=w2707:string)
              n2148 = String Subset(string=w2698, offset (0)=45, length (rest)=9 ("length (rest)")) -> (substring=w2713:string)
              n2149 = String Subset(string=w2698, offset (0)=65, length (rest)=9 ("length (rest)")) -> (substring=w2719:string)
              n2150 = Fract/Exp String To Number(string=w2705) -> (number=w2702:dbl)  [unwired: 3 in, 1 out]
              n2151 = Fract/Exp String To Number(string=w2699) -> (number=w2697:dbl)  [unwired: 3 in, 1 out]
              n2152 = Fract/Exp String To Number(string=w2707) -> (number=w2706:dbl)  [unwired: 3 in, 1 out]
              n2153 = Fract/Exp String To Number(string=w2713) -> (number=w2710:dbl)  [unwired: 3 in, 1 out]
              n2154 = Fract/Exp String To Number(string=w2719) -> (number=w2716:dbl)  [unwired: 3 in, 1 out]
              n2155 = Add(x=w2716, y=0.0) -> (x+y=w2714:dbl)
            }
            n2156 = for {
              N: w2568 -> [_]
              tunnel: w2579 -> [w2659]
              tunnel: w2578 -> [w2658]
              tunnel: [w2648] -> w2537 mode=indexing
              tunnel: [w2646] -> w2535 mode=indexing
              tunnel: [w2647] -> w2531 mode=indexing
              tunnel: w2566 -> [_]
              tunnel: [w2640] -> w2533 mode=indexing
              tunnel: [w2636] -> w2515 mode=indexing
              tunnel: [w2632] -> w2491 mode=indexing
              tunnel: [w2629] -> w2472 mode=indexing
              tunnel: [w2625] -> w2431 mode=indexing
              (unwired) 9 ("length (rest)")
              (unwired) 9 ("length (rest)")
              (unwired) TRUE ("line mode (F)")
              n2157 = Read from Text File "Read File"(file (use dialog)=w2658, error in=w2659) -> (text=w2626:string)  [unwired: 2 in, 3 out]
              n2158 = local write "String 8"(w2626) -> ()
              n2159 = String Subset(string=w2626, offset (0)=85) -> (substring=w2628:string)  [unwired: 1 in]
              n2160 = String Subset(string=w2626, offset (0)=35, length (rest)=9 ("length (rest)")) -> (substring=w2649:string)
              n2161 = String Subset(string=w2626, offset (0)=55, length (rest)=9 ("length (rest)")) -> (substring=w2634:string)
              n2162 = String Subset(string=w2626, offset (0)=25) -> (substring=w2630:string)  [unwired: 1 in]
              n2163 = String Subset(string=w2626, offset (0)=15, length (rest)=9 ("length (rest)")) -> (substring=w2655:string)
              n2164 = String Subset(string=w2626, offset (0)=0, length (rest)=14 ("length (rest)")) -> (substring=w2652:string)
              n2165 = String Subset(string=w2626, offset (0)=45, length (rest)=9 ("length (rest)")) -> (substring=w2639:string)
              n2166 = String Subset(string=w2626, offset (0)=65, length (rest)=9 ("length (rest)")) -> (substring=w2645:string)
              n2167 = Fract/Exp String To Number(string=w2628) -> (number=w2625:dbl)  [unwired: 3 in, 1 out]
              n2168 = Fract/Exp String To Number(string=w2649) -> (number=w2647:dbl)  [unwired: 3 in, 1 out]
              n2169 = Fract/Exp String To Number(string=w2634) -> (number=w2632:dbl)  [unwired: 3 in, 1 out]
              n2170 = Fract/Exp String To Number(string=w2630) -> (number=w2629:dbl)  [unwired: 3 in, 1 out]
              n2171 = Fract/Exp String To Number(string=w2655) -> (number=w2646:dbl)  [unwired: 3 in, 1 out]
              n2172 = Fract/Exp String To Number(string=w2652) -> (number=w2648:dbl)  [unwired: 3 in, 1 out]
              n2173 = Fract/Exp String To Number(string=w2639) -> (number=w2636:dbl)  [unwired: 3 in, 1 out]
              n2174 = Fract/Exp String To Number(string=w2645) -> (number=w2642:dbl)  [unwired: 3 in, 1 out]
              n2175 = Add(x=w2642, y=0.0) -> (x+y=w2640:dbl)
            }
            n2176 = String To Path(string=w2485) -> (path=w2583:path)
            n2177 = String To Path(string=w2483) -> (path=w2577:path)
            n2178 = local read "Numeric 11"() -> (w2567:i32)
            n2179 = local read "Numeric 13"() -> (w2569:i32)
            n2180 = Open/Create/Replace File "Open File"(file path (use dialog)=w2583) -> (refnum out=w2581:refnum<file>, error out=w2580:errorcluster)  [unwired: 5 in, 1 out]
            n2181 = Open/Create/Replace File "Open File"(file path (use dialog)=w2577) -> (refnum out=w2576:refnum<file>, error out=w2575:errorcluster)  [unwired: 5 in, 1 out]
            n2182 = for {
              N: w2567 -> [_]
              tunnel: w2581 -> [w2696]
              tunnel: w2580 -> [w2695]
              tunnel: [w2685] -> w2547 mode=indexing
              tunnel: [w2683] -> w2545 mode=indexing
              tunnel: [w2684] -> w2540 mode=indexing
              tunnel: w2566 -> [_]
              tunnel: [w2677] -> w2542 mode=indexing
              tunnel: [w2673] -> w2518 mode=indexing
              tunnel: [w2669] -> w2493 mode=indexing
              tunnel: [w2665] -> w2474 mode=indexing
              tunnel: [w2660] -> w2432 mode=indexing
              (unwired) TRUE ("line mode (F)")
              n2183 = Read from Text File "Read File"(file (use dialog)=w2696, error in=w2695) -> (text=w2661:string)  [unwired: 2 in, 3 out]
              n2184 = local write "String 7"(w2661) -> ()
              n2185 = String Subset(string=w2661, offset (0)=85, length (rest)=9 ("length (rest)")) -> (substring=w2664:string)
              n2186 = String Subset(string=w2661, offset (0)=35, length (rest)=9 ("length (rest)")) -> (substring=w2686:string)
              n2187 = String Subset(string=w2661, offset (0)=55, length (rest)=9 ("length (rest)")) -> (substring=w2672:string)
              n2188 = String Subset(string=w2661, offset (0)=25, length (rest)=9 ("length (rest)")) -> (substring=w2666:string)
              n2189 = String Subset(string=w2661, offset (0)=45, length (rest)=9 ("length (rest)")) -> (substring=w2674:string)
              n2190 = String Subset(string=w2661, offset (0)=0, length (rest)=14 ("length (rest)")) -> (substring=w2689:string)
              n2191 = String Subset(string=w2661, offset (0)=15, length (rest)=9 ("length (rest)")) -> (substring=w2692:string)
              n2192 = String Subset(string=w2661, offset (0)=65, length (rest)=9 ("length (rest)")) -> (substring=w2678:string)
              n2193 = Fract/Exp String To Number(string=w2664) -> (number=w2660:dbl)  [unwired: 3 in, 1 out]
              n2194 = Fract/Exp String To Number(string=w2686) -> (number=w2684:dbl)  [unwired: 3 in, 1 out]
              n2195 = Fract/Exp String To Number(string=w2672) -> (number=w2669:dbl)  [unwired: 3 in, 1 out]
              n2196 = Fract/Exp String To Number(string=w2666) -> (number=w2665:dbl)  [unwired: 3 in, 1 out]
              n2197 = Fract/Exp String To Number(string=w2674) -> (number=w2673:dbl)  [unwired: 3 in, 1 out]
              n2198 = Fract/Exp String To Number(string=w2689) -> (number=w2685:dbl)  [unwired: 3 in, 1 out]
              n2199 = Fract/Exp String To Number(string=w2692) -> (number=w2683:dbl)  [unwired: 3 in, 1 out]
              n2200 = Fract/Exp String To Number(string=w2678) -> (number=w2681:dbl)  [unwired: 3 in, 1 out]
              n2201 = Add(x=w2681, y=0.0) -> (x+y=w2677:dbl)
            }
            n2202 = for {
              N: w2569 -> [_]
              tunnel: w2576 -> [w2624]
              tunnel: w2575 -> [w2623]
              tunnel: [w2613] -> w2529 mode=indexing
              tunnel: [w2612] -> w2522 mode=indexing
              tunnel: w2566 -> [_]
              tunnel: [w2601] -> w2527 mode=indexing
              tunnel: [w2606] -> w2524 mode=indexing
              tunnel: [w2602] -> w2514 mode=indexing
              tunnel: [w2597] -> w2489 mode=indexing
              tunnel: [w2593] -> w2470 mode=indexing
              tunnel: [w2588] -> w2430 mode=indexing
              (unwired) 1.0 ("x")
              (unwired) TRUE ("line mode (F)")
              n2203 = Read from Text File "Read File"(file (use dialog)=w2624, error in=w2623) -> (text=w2589:string)  [unwired: 2 in, 3 out]
              n2204 = local write "String 12"(w2589) -> ()
              n2205 = String Subset(string=w2589, offset (0)=85, length (rest)=9 ("length (rest)")) -> (substring=w2591:string)
              n2206 = String Subset(string=w2589, offset (0)=35, length (rest)=9 ("length (rest)")) -> (substring=w2614:string)
              n2207 = String Subset(string=w2589, offset (0)=55, length (rest)=9 ("length (rest)")) -> (substring=w2599:string)
              n2208 = String Subset(string=w2589, offset (0)=25, length (rest)=9 ("length (rest)")) -> (substring=w2595:string)
              n2209 = String Subset(string=w2589, offset (0)=45, length (rest)=9 ("length (rest)")) -> (substring=w2604:string)
              n2210 = String Subset(string=w2589, offset (0)=15, length (rest)=9 ("length (rest)")) -> (substring=w2620:string)
              n2211 = String Subset(string=w2589, offset (0)=0, length (rest)=14 ("length (rest)")) -> (substring=w2617:string)
              n2212 = String Subset(string=w2589, offset (0)=65, length (rest)=9 ("length (rest)")) -> (substring=w2607:string)
              n2213 = Fract/Exp String To Number(string=w2591) -> (number=w2588:dbl)  [unwired: 3 in, 1 out]
              n2214 = Fract/Exp String To Number(string=w2614) -> (number=w2612:dbl)  [unwired: 3 in, 1 out]
              n2215 = Fract/Exp String To Number(string=w2599) -> (number=w2597:dbl)  [unwired: 3 in, 1 out]
              n2216 = Fract/Exp String To Number(string=w2595) -> (number=w2593:dbl)  [unwired: 3 in, 1 out]
              n2217 = Fract/Exp String To Number(string=w2604) -> (number=w2602:dbl)  [unwired: 3 in, 1 out]
              n2218 = Fract/Exp String To Number(string=w2620) -> (number=w2601:dbl)  [unwired: 3 in, 1 out]
              n2219 = Fract/Exp String To Number(string=w2617) -> (number=w2613:dbl)  [unwired: 3 in, 1 out]
              n2220 = Fract/Exp String To Number(string=w2607) -> (number=w2610:dbl)  [unwired: 3 in, 1 out]
              n2221 = Add(x=w2610, y=0.0) -> (x+y=w2606:dbl)
            }
            n2222 = Delete From Array(array=w2472, index=0) -> (array with subset deleted=w2445:dbl[])  [unwired: 1 in, 1 out]
            n2223 = Delete From Array(array=w2535, index=0) -> (array with subset deleted=w2508:dbl[])  [unwired: 1 in, 1 out]
            n2224 = Delete From Array(array=w2515, index=0) -> (array with subset deleted=w2503:dbl[])  [unwired: 1 in, 1 out]
            n2225 = Delete From Array(array=w2533, index=0) -> (array with subset deleted=w2534:dbl[])  [unwired: 1 in, 1 out]